vi "cameraCalibration.vi"() -> ()   [LabVIEW 2020]
uses:
  <vilib>/userDefined/High Color/IMAQdx.ctl
  controls/StateMachineVariables.ctl
  <vilib>/vision/Avi.llb/IMAQ AVI2 Refnum.ctl
  <vilib>/vision/Deep Learning.llb/IMAQ DL Model Refnum.ctl
  <vilib>/vision/Image Controls.llb/IMAQ Image.ctl
  <vilib>/Utility/file.llb/Write Delimited Spreadsheet (string).vi
panel:
  in  "Cancel":bool
  in  "input cluster":T1
  in  "Recalibrate":bool
  in  "Calibration mode":enum32{"Automatic detection", "Manual input"}(tab)
  out "Analyzed Image":T2(plugin-control)
  in  "Car side":enum32{"Item 0", "Item 1"}(radio)
  in  "Camera height (m)":dbl=1.36
  in  "Lateral y distance (m)":dbl=-1.03
  in  "Longitudinal x distance (m)":dbl=7.03
  in  "grab/resume":bool
  in  "Select camera":T3="cam0"
  in  "Video width":i32=1920
  in  "Video height":i32=1080
  in  "Video:rotate":bool
  in  "Lateral y distance (m)":dbl=-1.03
  in  "Longitudinal x distance (m)":dbl=7.03
  in  "Image x coordinate (px)":dbl=1179.0
  in  "Image y coordinate (px)":dbl=800.0
  in  "Camera height (m)":dbl=1.36
  in  "Image height (px)":dbl=1080.0
  in  "Image width (px)":dbl=1920.0
  # "To provide obstacle position information, the detection software needs 1) height of the camera above ground and 2) real and pixel coordinates of one arbitrary point in the view 3) pixel dimensions of the image (width and height). \n\nCamera calibration can be done either in Manual or Automatic mode: \n\nIn Manual Input mode, both pixel and real coordinate values need to be plugged in, using a snapped image from the camera and finding the pixel values of such point manually.\n\nIn Automatic Detection mode, the program can automatically detect a vehicle and obtain its pixel coordinates and therefore only real coordinates need to be plugged in.\n\nThe camera height needs to be plugged in in both modes.\n\nThe width and height values in manual mode are the dimensions of the used image, whereas in automatic mode, they can be set to an arbitrary value and the program will obtain pixel coordinates accordingly. As long as the aspect ratio of the calibration image is the same as the one used later for detection, the absolute pixel values of the calibration image do not matter (e. g. 1280x720 can be used instead of 1920x1080).\n\nThe camera is properly aligned when the horizon is vertically in the middle of the image."
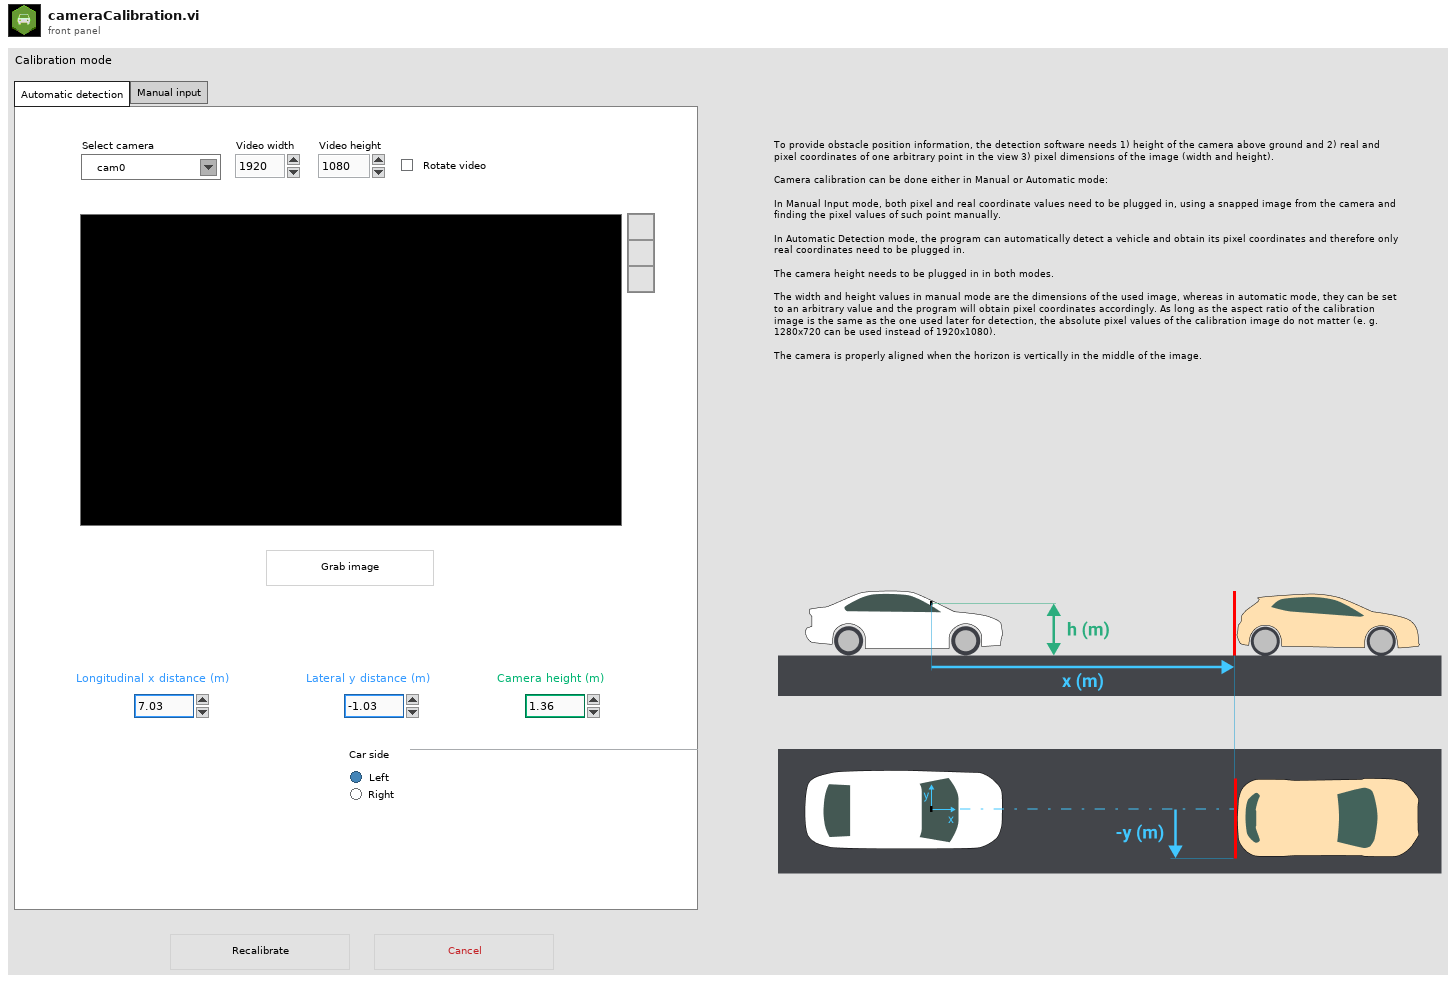
[diagram p1: front panel]
types:
  T1 = cluster{"Camera height (m)":dbl, "Longitudinal x distance (m)":dbl, "Lateral y distance (m)":dbl, "Image y coordinate (px)":dbl, "Image x coordinate (px)":dbl, "Image height (px)":i16, "Image width (px)":i16}
  T2 = typedef "IMAQ Image.ctl" = refnum<image>
  T3 = typedef "IMAQdx.ctl" = refnum<k21>
  T4 = enum32{"invalid app kind", "Development System", "Run Time System", "Student Edition", "Embedded LabVIEW", "Evaluation", "Custom"}
  T5 = typedef "StateMachineVariables.ctl" = cluster{"AVI Refnum":T6, "Session ID":T3, "TensorFlow model refnum":T7, "Image refnum":T2, "Longitudinal distance (m)":dbl, "Lateral distance (m)":dbl, "Relative speed (m/s)":dbl, "FPS":dbl, "Speed (km/h)":dbl, "Frame multiplier":u32, "Calibration: F_x":dbl, "Calibration: F_y":dbl, "Calibration: h (m)":dbl, "Video:width [px]":i32, "Video:heigth [px]":i32, "Video:rotate":bool}
  T6 = typedef "IMAQ AVI2 Refnum.ctl" = refnum<k20>
  T7 = typedef "IMAQ DL Model Refnum.ctl" = refnum<k20>
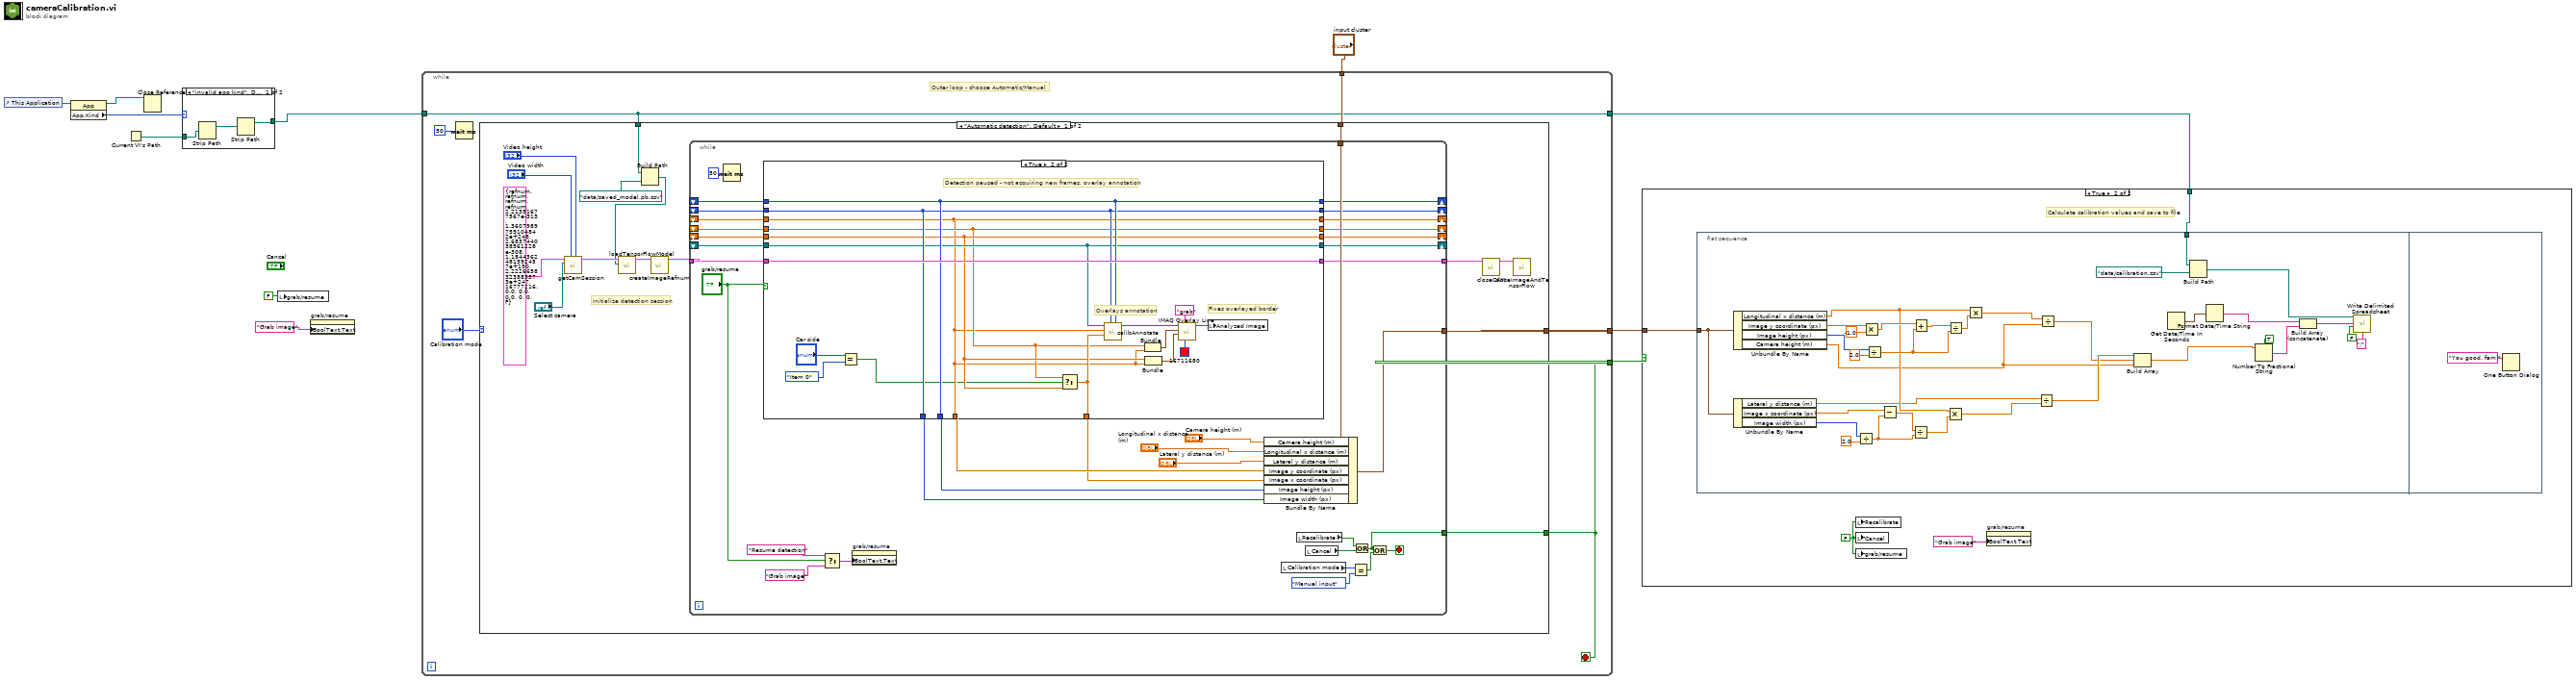
[diagram p0: block diagram]
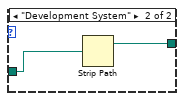
[diagram p2: hidden frame]
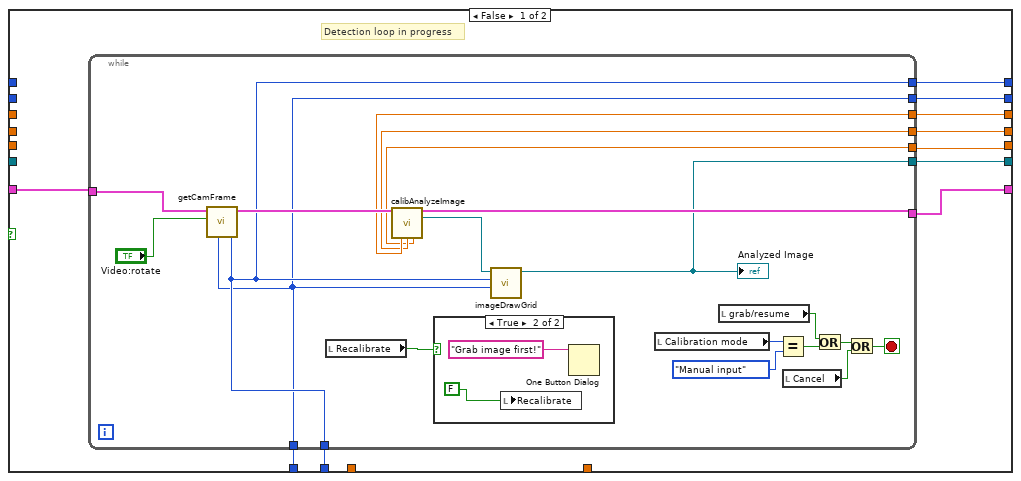
[diagram p4: hidden frame]
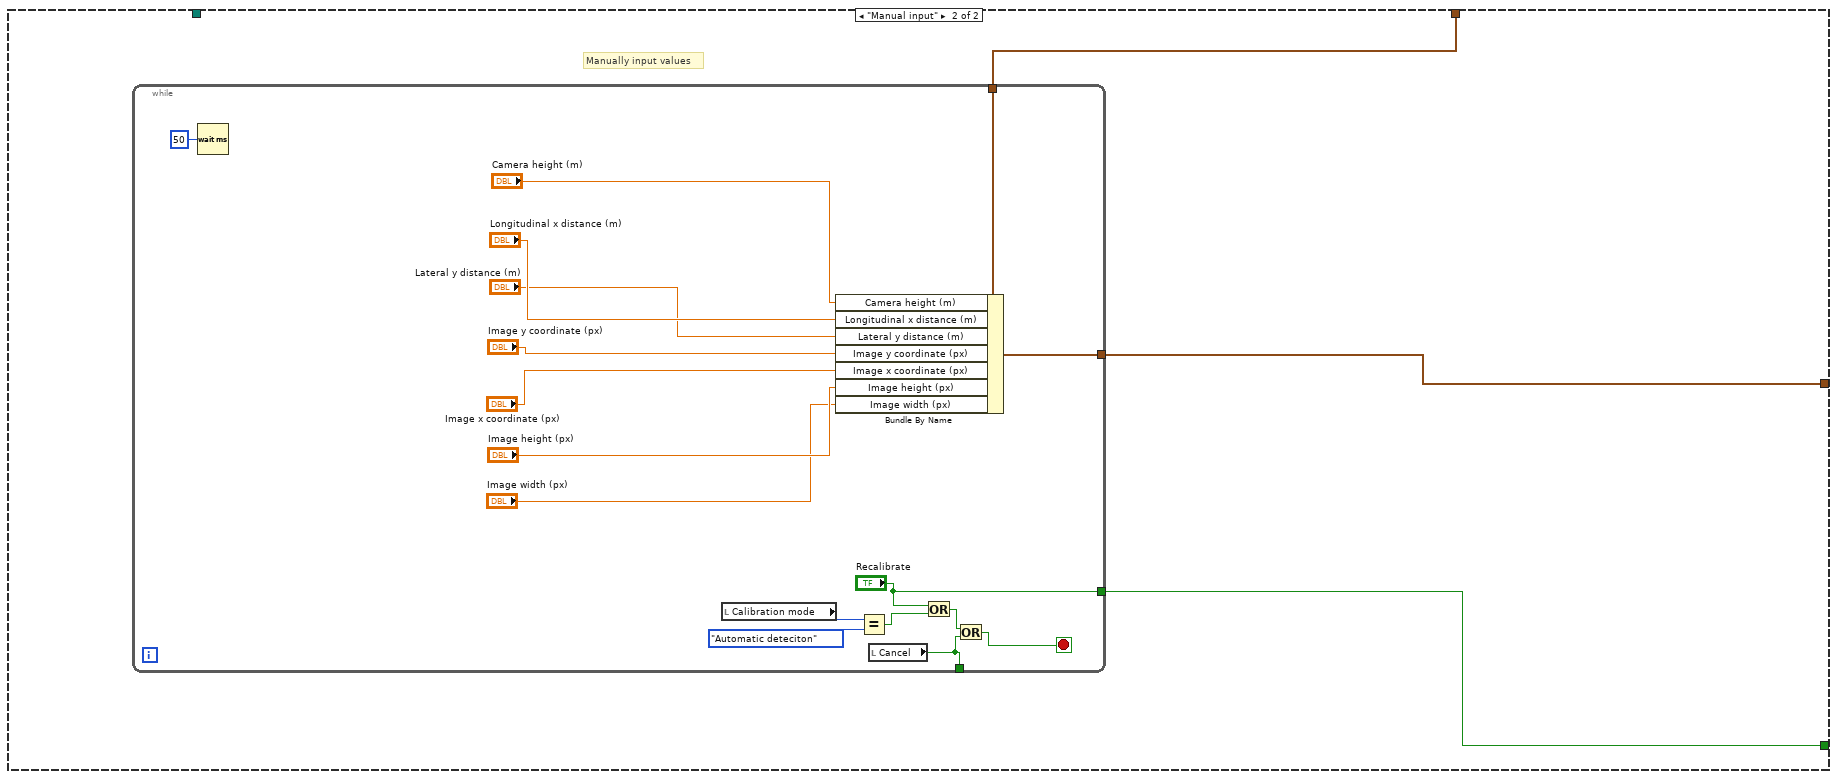
[diagram p6: hidden frame]
diagram:
  n1 = control-ref of="This Application"() -> (w6:refnum<vi>)
  n2 = property class="App"(reference=w6) -> (reference out=w5:refnum<vi>, "App.Kind"=w4:T4)  [unwired: 1 in, 1 out]
  n3 = Current VI's Path() -> (path=w3:path)
  n4 = Close Reference(reference=w5) -> ()  [unwired: 1 in, 1 out]
  n5 = case shown="\"invalid app kind\", Default" w4 {
    tunnel: w3 -> [w14 w16]
    tunnel: [w12 w15] -> w2
    frame "invalid app kind", Default {
      n6 = Strip Path(path=w14) -> (stripped path=w13:path)  [unwired: 1 out]
      n7 = Strip Path(path=w13) -> (stripped path=w12:path)  [unwired: 1 out]
    }
    frame "Development System" {
      n8 = Strip Path(path=w16) -> (stripped path=w15:path)  [unwired: 1 out]
    }
  }
  n9 = local write "grab/resume"(FALSE ("grab/resume")) -> ()
  n10 = property on="grab/resume" class="Bool (strict)"("BoolText.Text"="Grab image") -> ()  [unwired: 2 in, 2 out]
  n11 = while {
    tunnel: [w17] -> w11
    tunnel: [w20] -> w10
    tunnel: "input cluster" -> [w19]
    tunnel: w2 -> [w18]
    tunnel: [w18] -> w1
    stop <- w17 stop-if-true
    # "Outer loop - choose Automatic/Manual"
    n12 = Wait (ms)(milliseconds to wait=u32 50) -> ()  [unwired: 1 out]
    n13 = case shown="\"Automatic detection\", Default" "Calibration mode" {
      tunnel: [w37 w123] -> w17
      tunnel: [w35 w122] -> w20
      tunnel: w19 -> [w36 w121]
      tunnel: w18 -> [w24 _]
      frame "Automatic detection", Default {
        # "Initialize detection session"
        n14 = call "getCamSession.vi"("Video:heigth [px]"="Video height", "Video:width [px]"="Video width", "Session In"="Select camera", "Input cluster"=T5 {"AVI Refnum"=refnum, "Session ID"="", "TensorFlow model refnum"=refnum, "Image refnum"=refnum, "Longitudinal distance (m)"=0.0, "Lateral distance (m)"=0.0, "Relative speed (m/s)"=0.0, "FPS"=0.0, "Speed (km/h)"=0.0, "Frame multiplier"=0, "Calibration: F_x"=0.0, "Calibration: F_y"=0.0, "Calibration: h (m)"=0.0, "Video:width [px]"=0, "Video:heigth [px]"=0, "Video:rotate"=FALSE}) -> ("Output cluster"=w34:T5)  [unwired: 6 in, 1 out]
        n15 = Build Path(base path=w24, name or relative path=path "data/saved_model.pb.csv") -> (appended path=w23:path)
        n16 = call "loadTensorFlowModel.vi"("Path"=w23, "Input cluster"=w34) -> ("Output cluster"=w33:T5)  [unwired: 8 in, 1 out]
        n17 = call "createImageRefnum.vi"("Output cluster in"=w33) -> ("Output cluster out"=w31:T5)  [unwired: 9 in, 1 out]
        n18 = while {
          tunnel: [w42] -> w37
          tunnel: w36 -> [w66]
          tunnel: [w62] -> w35
          tunnel: w31 -> [w61]
          tunnel: [w60] -> w30
          shift-right: [w55] -> _
          shift-left: _ -> [w48]
          shift-right: [w54] -> _
          shift-left: _ -> [w47]
          shift-right: [w53] -> _
          shift-left: _ -> [w46]
          shift-right: [w52] -> _
          shift-left: _ -> [w51]
          shift-right: [w56] -> _
          shift-left: _ -> [w49]
          shift-right: [w57] -> _
          shift-left: _ -> [w50]
          stop <- w45 stop-if-true
          n19 = Wait (ms)(milliseconds to wait=u32 50) -> ()  [unwired: 1 out]
          n20 = case shown="True" "grab/resume" {
            tunnel: [w82 w119] -> w58
            tunnel: w61 -> [w81 w120]
            tunnel: [w80 w118] -> w59
            tunnel: [w79 w120] -> w60
            tunnel: [_ w107] -> w41
            tunnel: [w78 w119] -> w57
            tunnel: [w77 w118] -> w56
            tunnel: [w76 w107] -> w55
            tunnel: [w75 w108] -> w54
            tunnel: [w74 w109] -> w53
            tunnel: [w73 w117] -> w52
            tunnel: w51 -> [_ w117]
            tunnel: w50 -> [_ w119]
            tunnel: w49 -> [_ w118]
            tunnel: w48 -> [_ w107]
            tunnel: w47 -> [_ w108]
            tunnel: w46 -> [_ w109]
            tunnel: [_ w110] -> w40
            frame False {
              # "Detection loop in progress"
              n21 = while {
                tunnel: w81 -> [w97]
                tunnel: [w93] -> w82
                tunnel: [w92] -> w80
                tunnel: [w95] -> w79
                tunnel: [w93] -> w78
                tunnel: [w92] -> w77
                tunnel: [w91] -> w76
                tunnel: [w90] -> w75
                tunnel: [w89] -> w74
                tunnel: [w88] -> w73
                stop <- w87 stop-if-true
                n22 = call "getCamFrame.vi"("Video:rotate"="Video:rotate", "Cluster"=w97) -> ("output cluster"=w96:T5, "Image height"=w93:i32, "Image width"=w92:i32)  [unwired: 5 in, 2 out]
                n23 = local read "Recalibrate"() -> (w83:bool)
                n24 = call "calibAnalyzeImage.vi"("Input cluster"=w96) -> ("Output cluster"=w95:T5, "Image out"=w94:T2, "bottom border"=w91:sgl, "left border"=w90:sgl, "right border"=w89:sgl)  [unwired: 9 in, 1 out]
                n25 = case shown="True" w83 {
                  frame False {
                  }
                  frame True {
                    n26 = local write "Recalibrate"(FALSE ("Recalibrate")) -> ()
                    n27 = One Button Dialog(message="Grab image first!") -> ()  [unwired: 1 in, 1 out]
                  }
                }
                n28 = call "imageDrawGrid.vi"("Image"=w94, "Image height"=w93, "Image width"=w92) -> ("Image Out"=w88:T2)  [unwired: 7 in]
                "Analyzed Image" <- w88
                n29 = local read "Calibration mode"() -> (w101:enum32{"Automatic detection", "Manual input"})
                n30 = local read "grab/resume"() -> (w98:bool)
                n31 = Equal?(x=w101, y=enum32{"Automatic detection", "Manual input"}."Manual input") -> (x = y?=w99:bool)
                n32 = local read "Cancel"() -> (w86:bool)
                n33 = Or(x=w98, y=w99) -> (x .or. y?=w85:bool)
                n34 = Or(x=w85, y=w86) -> (x .or. y?=w87:bool)
              }
            }
            frame True {
              # "Overlays annotation"
              # "Fixes overlayed border"
              # "Detection paused - not acquiring new frames, overlay annotation"
              n35 = Equal?(x="Car side", y=enum32{"Item 0", "Item 1"}."Item 0") -> (x = y?=w104:bool)
              n36 = Select(t=w108, s=w104, f=w109) -> (s? t:f=w110:sgl)
              n37 = call "calibAnnotate.vi"("Image height"=w119, "Image width"=w118, "Side border"=w110, "Bottom border"=w107, "Image"=w117) -> ("Image Out"=w116:T2)  [unwired: 6 in]
              n38 = Bundle("left border"=w108, "bottom border"=w107) -> (w114:cluster{"left border":sgl, "bottom border":sgl})  [unwired: 1 in]
              n39 = Bundle("right border"=w109, "bottom border"=w107) -> (w115:cluster{"right border":sgl, "bottom border":sgl})  [unwired: 1 in]
              n40 = call "IMAQ Overlay Line"("Color"=u32 16711680, "Group"="grab", "End Point"=w115, "Start Point"=w114, "Image"=w116) -> ("Image Out"=w112:T2)  [unwired: 5 in, 1 out]
              n41 = local write "Analyzed Image"(w112) -> ()
            }
          }
          n42 = Select(t="Resume detection", s="grab/resume", f="Grab image") -> (s? t:f=w69:string)
          n43 = property on="grab/resume" class="Bool (strict)"("BoolText.Text"=w69) -> ()  [unwired: 2 in, 2 out]
          n44 = Bundle By Name(cluster=w66, "Camera height (m)"="Camera height (m)", "Longitudinal x distance (m)"="Longitudinal x distance (m)", "Lateral y distance (m)"="Lateral y distance (m)", "Image y coordinate (px)"=w41, "Image x coordinate (px)"=w40, "Image height (px)"=w58, "Image width (px)"=w59) -> (w62:T1)
          n45 = local read "Calibration mode"() -> (w71:enum32{"Automatic detection", "Manual input"})
          n46 = local read "Recalibrate"() -> (w38:bool)
          n47 = local read "Cancel"() -> (w44:bool)
          n48 = Equal?(x=w71, y=enum32{"Automatic deteciton", "Manual input"}."Manual input") -> (x = y?=w43:bool)
          n49 = Or(x=w38, y=w44) -> (x .or. y?=w42:bool)
          n50 = Or(x=w42, y=w43) -> (x .or. y?=w45:bool)
        }
        n51 = call "closeCAM.vi"("Input cluster"=w30) -> ("Output cluster"=w29:T5)  [unwired: 9 in, 1 out]
        n52 = call "closeImageAndTensorFlow.vi"("Input cluster"=w29) -> ()  [unwired: 9 in, 2 out]
      }
      frame "Manual input" {
        # "Manually input values"
        n53 = while {
          tunnel: ["Recalibrate"] -> w123
          tunnel: [w127] -> w122
          tunnel: w121 -> [w135]
          tunnel: [w124] -> _
          stop <- w125 stop-if-true
          n54 = Wait (ms)(milliseconds to wait=u32 50) -> ()  [unwired: 1 out]
          n55 = local read "Calibration mode"() -> (w140:enum32{"Automatic detection", "Manual input"})
          n56 = Bundle By Name(cluster=w135, "Camera height (m)"="Camera height (m)", "Longitudinal x distance (m)"="Longitudinal x distance (m)", "Lateral y distance (m)"="Lateral y distance (m)", "Image y coordinate (px)"="Image y coordinate (px)", "Image x coordinate (px)"="Image x coordinate (px)", "Image height (px)"="Image height (px)", "Image width (px)"="Image width (px)") -> (w127:T1)
          n57 = Equal?(x=w140, y=enum32{"Automatic deteciton", "Manual input"}."Automatic deteciton") -> (x = y?=w137:bool)
          n58 = local read "Cancel"() -> (w124:bool)
          n59 = Or(x="Recalibrate", y=w137) -> (x .or. y?=w126:bool)
          n60 = Or(x=w126, y=w124) -> (x .or. y?=w125:bool)
        }
      }
    }
  }
  n61 = case shown="True" w11 {
    tunnel: w10 -> [_ w144]
    tunnel: w1 -> [_ w143]
    frame False {
    }
    frame True {
      w141 = FALSE ("Recalibrate")
      # "Calculate calibration values and save to file"
      n62 = flat-sequence {
        tunnel: w144 -> [w176]
        tunnel: w143 -> [w146]
        frame #0 {
          n63 = Unbundle By Name(w176) -> ("Longitudinal x distance (m)"=w161:dbl, "Image y coordinate (px)"=w175:dbl, "Image height (px)"=w172:i16, "Camera height (m)"=w156:dbl)
          n64 = Unbundle By Name(w176) -> ("Lateral y distance (m)"=w159:dbl, "Image x coordinate (px)"=w163:dbl, "Image width (px)"=w166:i16)
          n65 = Divide(x=w166, y=2.0) -> (x/y=w164:dbl)
          n66 = Multiply(x=w175, y=-1.0) -> (x*y=w173:dbl)
          n67 = Divide(x=w172, y=2.0) -> (x/y=w170:dbl)
          n68 = Subtract(x=w163, y=w164) -> (x-y=w165:dbl)
          n69 = Divide(x=w165, y=w164) -> (x/y=w162:dbl)
          n70 = Add(x=w173, y=w170) -> (x+y=w177:dbl)
          n71 = Multiply(x=w161, y=w162) -> (x*y=w160:dbl)
          n72 = Divide(x=w177, y=w170) -> (x/y=w169:dbl)
          n73 = Multiply(x=w161, y=w169) -> (x*y=w168:dbl)
          n74 = Divide(x=w159, y=w160) -> (x/y=w158:dbl)
          n75 = Divide(x=w168, y=w156) -> (x/y=w157:dbl)
          n76 = Build Array(w158, w157, w156) -> (w149:dbl[])
          n77 = Get Date/Time In Seconds() -> (seconds since 1Jan1904=w155:timestamp)
          n78 = Build Path(base path=w146, name or relative path=path "data/calibration.csv") -> (appended path=w145:path)
          n79 = Format Date/Time String(seconds (now)=w155) -> (date/time string=w148:string)  [unwired: 2 in]
          n80 = Number To Fractional String(use system decimal point (T)=TRUE, number=w149) -> (F-format string=w152:string[])  [unwired: 2 in]
          n81 = Build Array (concatenate)(w148, w152) -> (w151:string[])
          n82 = call-poly <vilib>:"Write Delimited Spreadsheet.vi"("file path (dialog if empty)"=w145, "1D data"=w151, "append to file? (new file:F)"=FALSE, "delimiter (\\t)"=";" ("delimiter (\\t)")) -> ()  [unwired: 10 in, 2 out]
        }
        frame #1 {
          n83 = One Button Dialog(message="You good, fam!") -> ()  [unwired: 1 in, 1 out]
        }
      }
      n84 = local write "Recalibrate"(w141) -> ()
      n85 = local write "Cancel"(w141) -> ()
      n86 = local write "grab/resume"(w141) -> ()
      n87 = property on="grab/resume" class="Bool (strict)"("BoolText.Text"="Grab image") -> ()  [unwired: 2 in, 2 out]
    }
  }
